vi "FlexMag - 23-03-2023.vi"() -> ()   [LabVIEW 2018] (continued)
                                frame True {
                                n21590 = Wait Until Next ms Multiple(millisecond multiple=u32 200) -> ()  [unwired: 1 out]
                                n21591 = local write "CH3_SoV_Ar_DO"(FALSE ("coating error")) -> ()
                                }
                                }
                                n21592 = local read "coating start"() -> (w25607:bool)
                                n21593 = local read "abort ch3"() -> (w25601:bool)
                                n21594 = Not(x=w25607) -> (.not. x?=w25606:bool)
                                n21595 = Compound Arithmetic op=OR(w25608, w25606, w25601) -> (w25605:bool)
                                }
                                }
                                }
                                }
                                frame True {
                                }
                                }
                                }
                                frame #1 {
                                n21596 = local read "abort ch3"() -> (w25615:bool)
                                n21597 = case shown="False" w25615 {
                                frame False {
                                n21598 = local read "coating start"() -> (w25616:bool)
                                n21599 = case shown="True" w25616 {
                                frame False {
                                }
                                frame True {
                                n21600 = Wait (ms)(milliseconds to wait=u32 100) -> ()  [unwired: 1 out]
                                "coating ch3 led 16" <- TRUE ("coating ch2 led 1")
                                }
                                }
                                }
                                frame True {
                                }
                                }
                                }
                                }
                                }
                                frame #17 {
                                # "BG BV close"
                                n21601 = stacked-sequence {
                                frame #0 {
                                n21602 = local read "abort ch3"() -> (w25619:bool)
                                n21603 = case shown="False" w25619 {
                                frame False {
                                n21604 = local read "coating start"() -> (w25620:bool)
                                n21605 = case shown="True" w25620 {
                                frame False {
                                }
                                frame True {
                                n21606 = while {
                                i -> [w25624]
                                stop <- w25626 stop-if-true
                                n21607 = Greater Or Equal?(x=w25624, y=100) -> (x >= y?=w25625:bool)
                                n21608 = case shown="True" w25625 {
                                frame False {
                                }
                                frame True {
                                n21609 = local write "Warning Message"("Automatic Coating Process is canceled !\nCH3 BG BV couldn't be closed..." ("Warning Message")) -> ()
                                n21610 = local write "coating error"(TRUE ("coating error")) -> ()
                                }
                                }
                                n21611 = local read "CH3_BG_BV_DI"() -> (w25621:bool)
                                n21612 = case shown="True" w25621 {
                                tunnel: [TRUE ("CH2_WFC_DO") FALSE ("CH2_WFC_DO")] -> w25629
                                frame False {
                                }
                                frame True {
                                n21613 = Wait Until Next ms Multiple(millisecond multiple=u32 200) -> ()  [unwired: 1 out]
                                n21614 = local write "CH3_BG_BV_DO"(FALSE ("coating error")) -> ()
                                }
                                }
                                n21615 = local read "coating start"() -> (w25628:bool)
                                n21616 = local read "abort ch3"() -> (w25622:bool)
                                n21617 = Not(x=w25628) -> (.not. x?=w25627:bool)
                                n21618 = Compound Arithmetic op=OR(w25629, w25627, w25622) -> (w25626:bool)
                                }
                                }
                                }
                                }
                                frame True {
                                }
                                }
                                }
                                frame #1 {
                                n21619 = local read "abort ch3"() -> (w25636:bool)
                                n21620 = case shown="False" w25636 {
                                frame False {
                                n21621 = local read "coating start"() -> (w25637:bool)
                                n21622 = case shown="True" w25637 {
                                frame False {
                                }
                                frame True {
                                n21623 = Wait (ms)(milliseconds to wait=u32 100) -> ()  [unwired: 1 out]
                                "coating ch3 led 17" <- TRUE ("coating ch2 led 1")
                                }
                                }
                                }
                                frame True {
                                }
                                }
                                }
                                }
                                }
                                frame #18 {
                                # "CC open"
                                n21624 = stacked-sequence {
                                frame #0 {
                                n21625 = local read "abort ch3"() -> (w25640:bool)
                                n21626 = case shown="False" w25640 {
                                frame False {
                                n21627 = local read "coating start"() -> (w25641:bool)
                                n21628 = case shown="True" w25641 {
                                frame False {
                                }
                                frame True {
                                n21629 = while {
                                i -> [w25645]
                                stop <- w25647 stop-if-true
                                n21630 = Greater Or Equal?(x=w25645, y=100) -> (x >= y?=w25646:bool)
                                n21631 = case shown="True" w25646 {
                                frame False {
                                }
                                frame True {
                                n21632 = local write "Warning Message"("Automatic Coating Process is canceled !\nCH3 CC couldn't be opened..." ("Warning Message")) -> ()
                                n21633 = local write "coating error"(TRUE ("coating error")) -> ()
                                }
                                }
                                n21634 = local read "CH3_CC_DI"() -> (w25642:bool)
                                n21635 = case shown="False" w25642 {
                                tunnel: [FALSE ("CH2_WFC_DO") TRUE ("CH2_WFC_DO")] -> w25650
                                frame False {
                                n21636 = Wait Until Next ms Multiple(millisecond multiple=u32 200) -> ()  [unwired: 1 out]
                                n21637 = local write "CH3_CC_DO"(TRUE ("coating error")) -> ()
                                }
                                frame True {
                                }
                                }
                                n21638 = local read "coating start"() -> (w25649:bool)
                                n21639 = local read "abort ch3"() -> (w25643:bool)
                                n21640 = Not(x=w25649) -> (.not. x?=w25648:bool)
                                n21641 = Compound Arithmetic op=OR(w25650, w25648, w25643) -> (w25647:bool)
                                }
                                }
                                }
                                }
                                frame True {
                                }
                                }
                                }
                                frame #1 {
                                n21642 = local read "abort ch3"() -> (w25657:bool)
                                n21643 = case shown="False" w25657 {
                                frame False {
                                n21644 = local read "coating start"() -> (w25658:bool)
                                n21645 = case shown="True" w25658 {
                                frame False {
                                }
                                frame True {
                                n21646 = Wait (ms)(milliseconds to wait=u32 100) -> ()  [unwired: 1 out]
                                "coating ch3 led 18" <- TRUE ("coating ch2 led 1")
                                }
                                }
                                }
                                frame True {
                                }
                                }
                                }
                                }
                                }
                                frame #19 {
                                # "water close"
                                n21647 = stacked-sequence {
                                frame #0 {
                                n21648 = local read "abort ch3"() -> (w25661:bool)
                                n21649 = case shown="False" w25661 {
                                frame False {
                                n21650 = local read "coating start"() -> (w25662:bool)
                                n21651 = case shown="True" w25662 {
                                frame False {
                                }
                                frame True {
                                n21652 = while {
                                i -> [w25666]
                                stop <- w25668 stop-if-true
                                n21653 = Greater Or Equal?(x=w25666, y=100) -> (x >= y?=w25667:bool)
                                n21654 = case shown="True" w25667 {
                                frame False {
                                }
                                frame True {
                                n21655 = local write "Warning Message"("Automatic Coating Process is canceled !\nCH3 Water Flow couldn't be closed..." ("Warning Message")) -> ()
                                n21656 = local write "coating error"(TRUE ("coating error")) -> ()
                                }
                                }
                                n21657 = local read "CH3_WFC_DI"() -> (w25663:bool)
                                n21658 = case shown="True" w25663 {
                                tunnel: [TRUE ("CH2_WFC_DO") FALSE ("CH2_WFC_DO")] -> w25671
                                frame False {
                                }
                                frame True {
                                n21659 = Wait Until Next ms Multiple(millisecond multiple=u32 200) -> ()  [unwired: 1 out]
                                n21660 = local write "CH3_WFC_DO"(FALSE ("coating error")) -> ()
                                }
                                }
                                n21661 = local read "coating start"() -> (w25670:bool)
                                n21662 = local read "abort ch3"() -> (w25664:bool)
                                n21663 = Not(x=w25670) -> (.not. x?=w25669:bool)
                                n21664 = Compound Arithmetic op=OR(w25671, w25669, w25664) -> (w25668:bool)
                                }
                                }
                                }
                                }
                                frame True {
                                }
                                }
                                }
                                frame #1 {
                                n21665 = local read "abort ch3"() -> (w25678:bool)
                                n21666 = case shown="False" w25678 {
                                frame False {
                                n21667 = local read "coating start"() -> (w25679:bool)
                                n21668 = case shown="True" w25679 {
                                frame False {
                                }
                                frame True {
                                n21669 = Wait (ms)(milliseconds to wait=u32 100) -> ()  [unwired: 1 out]
                                "coating ch3 led 19" <- TRUE ("coating ch2 led 1")
                                }
                                }
                                }
                                frame True {
                                }
                                }
                                }
                                }
                                }
                                frame #20 {
                                # "back roll"
                                n21670 = stacked-sequence {
                                frame #0 {
                                n21671 = local read "abort ch3"() -> (w25682:bool)
                                n21672 = case shown="False" w25682 {
                                frame False {
                                n21673 = local read "coating start"() -> (w25683:bool)
                                n21674 = case shown="True" w25683 {
                                frame False {
                                }
                                frame True {
                                n21675 = disable-structure shown="Enabled" {
                                frame Disabled {
                                n21676 = flat-sequence {
                                frame #0 {
                                n21677 = local read "R DC number steps"() -> (w25684:dbl)
                                n21678 = local write "back roll"(TRUE ("back roll")) -> ()
                                n21679 = local write "step count"(w25684) -> ()
                                }
                                frame #1 {
                                n21680 = Wait (ms)(milliseconds to wait=u32 1000) -> ()  [unwired: 1 out]
                                }
                                frame #2 {
                                n21681 = while {
                                i -> [w25689]
                                stop <- w25695 stop-if-true
                                n21682 = local read "coating start"() -> (w25692:bool)
                                n21683 = local read "back roll"() -> (w25691:bool)
                                n21684 = local read "abort ch3"() -> (w25694:bool)
                                n21685 = Greater?(x=w25689, y=2000) -> (0:w25687:bool)
                                n21686 = local write "coating error"(w25687) -> ()
                                n21687 = Not(x=w25691) -> (.not. x?=w25690:bool)
                                n21688 = Not(x=w25692) -> (.not. x?=w25696:bool)
                                n21689 = Compound Arithmetic op=OR(w25690, w25696, w25694) -> (w25695:bool)
                                n21690 = Wait Until Next ms Multiple(millisecond multiple=u32 200) -> ()  [unwired: 1 out]
                                }
                                }
                                }
                                }
                                frame Enabled {
                                n21691 = local read "dep. for?"() -> (w25698:bool)
                                n21692 = Not(x=w25698) -> (.not. x?=w25699:bool)
                                n21693 = Wait (ms)(milliseconds to wait=u32 100) -> ()  [unwired: 1 out]
                                n21694 = local write "dep. for?"(w25699) -> ()
                                }
                                }
                                }
                                }
                                }
                                frame True {
                                }
                                }
                                }
                                frame #1 {
                                n21695 = local read "abort ch3"() -> (w25700:bool)
                                n21696 = case shown="False" w25700 {
                                frame False {
                                n21697 = local read "coating start"() -> (w25701:bool)
                                n21698 = case shown="True" w25701 {
                                frame False {
                                }
                                frame True {
                                n21699 = Wait (ms)(milliseconds to wait=u32 100) -> ()  [unwired: 1 out]
                                "coating ch3 led 20" <- TRUE ("coating ch2 led 1")
                                }
                                }
                                }
                                frame True {
                                }
                                }
                                }
                                }
                                }
                                frame #21 {
                                # "done"
                                n21700 = stacked-sequence {
                                frame #0 {
                                n21701 = local read "abort ch3"() -> (w25704:bool)
                                n21702 = case shown="False" w25704 {
                                frame False {
                                n21703 = local read "coating start"() -> (w25705:bool)
                                n21704 = case shown="True" w25705 {
                                frame False {
                                }
                                frame True {
                                n21705 = local write "Buzzer DO"(TRUE ("Buzzer DO")) -> ()
                                n21706 = Wait (ms)(milliseconds to wait=u32 3000) -> ()  [unwired: 1 out]
                                n21707 = local write "System Status"("COATING PROCESS DONE (CH3)" ("System Status")) -> ()
                                }
                                }
                                }
                                frame True {
                                }
                                }
                                }
                                frame #1 {
                                n21708 = local read "abort ch3"() -> (w25709:bool)
                                n21709 = case shown="False" w25709 {
                                frame False {
                                n21710 = local read "coating start"() -> (w25710:bool)
                                n21711 = case shown="True" w25710 {
                                frame False {
                                }
                                frame True {
                                n21712 = Wait (ms)(milliseconds to wait=u32 1000) -> ()  [unwired: 1 out]
                                n21713 = local write "System Status"("SEMI-AUTOMATIC MODE " ("System Status")) -> ()
                                n21714 = local write "Buzzer DO"(FALSE ("Buzzer DO")) -> ()
                                }
                                }
                                }
                                frame True {
                                }
                                }
                                }
                                }
                                }
                                }
                                }
                                }
                                }
                              }
                            }
                            frame "rfsputter" {
                              n21715 = disable-structure shown="Enabled" {
                                disable-tunnel: [w25715 TRUE] -> w25714
                                frame Disabled {
                                n21716 = local read "ch4 ch pg torr"() -> (w25720:dbl)
                                n21717 = local read "ch4 cc torr"() -> (w25721:dbl)
                                n21718 = Less Or Equal?(x=w25720, y=0.005) -> (x <= y?=w25719:bool)
                                n21719 = Less Or Equal?(x=w25721, y=0.005) -> (x <= y?=w25718:bool)
                                n21720 = And(x=w25719, y=w25718) -> (x .and. y?=w25715:bool)
                                }
                                frame Enabled {
                                }
                              }
                              n21721 = case shown="True" w25714 {
                                frame False {
                                n21722 = local write "coating error"(TRUE ("coating error")) -> ()
                                n21723 = local write "Warning Message"("Automatic Coating Process is canceled !\nCH4 Pressure should be under 5E-3 Torr .." ("Warning Message")) -> ()
                                }
                                frame True {
                                n21724 = stacked-sequence {
                                frame #0 {
                                }
                                frame #1 {
                                n21725 = stacked-sequence {
                                frame #0 {
                                n21726 = local read "abort ch4"() -> (w25725:bool)
                                n21727 = case shown="False" w25725 {
                                frame False {
                                n21728 = local read "coating start"() -> (w25726:bool)
                                n21729 = case shown="True" w25726 {
                                frame False {
                                }
                                frame True {
                                n21730 = local read "casette_ch4_gui"() -> (w25728:bool)
                                n21731 = Wait (ms)(milliseconds to wait=u32 100) -> ()  [unwired: 1 out]
                                n21732 = case shown="False" w25728 {
                                frame False {
                                n21733 = stacked-sequence {
                                frame #0 {
                                n21734 = flat-sequence {
                                frame #0 {
                                n21735 = local write "target chamber"(4.0 ("target chamber")) -> ()
                                n21736 = Wait (ms)(milliseconds to wait=u32 100) -> ()  [unwired: 1 out]
                                }
                                frame #1 {
                                n21737 = Wait (ms)(milliseconds to wait=u32 1000) -> ()  [unwired: 1 out]
                                }
                                frame #2 {
                                n21738 = local write "transfer vacuum auto"(TRUE ("transfer vacuum")) -> ()
                                }
                                }
                                }
                                frame #1 {
                                n21739 = while {
                                i -> [w25736]
                                stop <- w25738 stop-if-true
                                # "20min"
                                n21740 = local read "present location"() -> (w25742:dbl)
                                n21741 = local read "casette_ch4_gui"() -> (w25734:bool)
                                n21742 = local read "abort ch4"() -> (w25737:bool)
                                n21743 = Equal?(x=w25742, y=4.0) -> (x = y?=w25740:bool)
                                n21744 = Greater?(x=w25736, y=1200) -> (0:w25733:bool)
                                n21745 = local write "trns error"(w25733) -> ()
                                n21746 = Compound Arithmetic op=OR(w25737, w25740, w25734, w25733) -> (w25738:bool)
                                n21747 = Wait Until Next ms Multiple(millisecond multiple=u32 1000) -> ()  [unwired: 1 out]
                                }
                                }
                                }
                                }
                                frame True {
                                }
                                }
                                }
                                }
                                }
                                frame True {
                                }
                                }
                                }
                                frame #1 {
                                n21748 = local read "abort ch4"() -> (w25743:bool)
                                n21749 = case shown="False" w25743 {
                                frame False {
                                n21750 = local read "coating start"() -> (w25744:bool)
                                n21751 = case shown="True" w25744 {
                                frame False {
                                }
                                frame True {
                                n21752 = Wait (ms)(milliseconds to wait=u32 100) -> ()  [unwired: 1 out]
                                n21753 = local write "System Status"("COATING MODE ACTIVE" ("System Status")) -> ()
                                "coating ch4 led 1" <- TRUE ("coating ch2 led 1")
                                }
                                }
                                }
                                frame True {
                                }
                                }
                                }
                                }
                                }
                                frame #2 {
                                # "water"
                                n21754 = stacked-sequence {
                                frame #0 {
                                # "ch1 water off"
                                n21755 = local read "abort ch4"() -> (w25748:bool)
                                n21756 = case shown="False" w25748 {
                                frame False {
                                n21757 = local read "coating start"() -> (w25749:bool)
                                n21758 = case shown="True" w25749 {
                                frame False {
                                }
                                frame True {
                                n21759 = while {
                                i -> [w25752]
                                stop <- w25754 stop-if-true
                                n21760 = Greater Or Equal?(x=w25752, y=100) -> (x >= y?=w25753:bool)
                                n21761 = case shown="True" w25753 {
                                frame False {
                                }
                                frame True {
                                n21762 = local write "coating error"(TRUE ("coating error")) -> ()
                                n21763 = local write "Warning Message"("Automatic Coating Process is canceled !\nCH1 Water Flow Problem.." ("Warning Message")) -> ()
                                }
                                }
                                n21764 = local read "CH1_WFC_DI"() -> (w25758:bool)
                                n21765 = case shown="True" w25758 {
                                tunnel: [TRUE ("CH2_WFC_DO") FALSE ("CH2_WFC_DO")] -> w25757
                                frame False {
                                }
                                frame True {
                                n21766 = Wait Until Next ms Multiple(millisecond multiple=u32 200) -> ()  [unwired: 1 out]
                                n21767 = local write "CH1_WFC_DO"(FALSE ("CH2_WFC_DO")) -> ()
                                }
                                }
                                n21768 = local read "coating start"() -> (w25756:bool)
                                n21769 = local read "abort ch4"() -> (w25750:bool)
                                n21770 = Not(x=w25756) -> (.not. x?=w25755:bool)
                                n21771 = Compound Arithmetic op=OR(w25757, w25755, w25750) -> (w25754:bool)
                                }
                                }
                                }
                                }
                                frame True {
                                }
                                }
                                }
                                frame #1 {
                                # "ch3 water off"
                                n21772 = local read "abort ch4"() -> (w25765:bool)
                                n21773 = case shown="False" w25765 {
                                frame False {
                                n21774 = local read "coating start"() -> (w25766:bool)
                                n21775 = case shown="True" w25766 {
                                frame False {
                                }
                                frame True {
                                n21776 = while {
                                i -> [w25769]
                                stop <- w25771 stop-if-true
                                n21777 = Greater Or Equal?(x=w25769, y=100) -> (x >= y?=w25770:bool)
                                n21778 = case shown="True" w25770 {
                                frame False {
                                }
                                frame True {
                                n21779 = local write "coating error"(TRUE ("coating error")) -> ()
                                n21780 = local write "Warning Message"("Automatic Coating Process is canceled !\nCH3 Water Flow Problem.." ("Warning Message")) -> ()
                                }
                                }
                                n21781 = local read "CH3_WFC_DI"() -> (w25775:bool)
                                n21782 = case shown="True" w25775 {
                                tunnel: [TRUE ("CH2_WFC_DO") FALSE ("CH2_WFC_DO")] -> w25774
                                frame False {
                                }
                                frame True {
                                n21783 = Wait Until Next ms Multiple(millisecond multiple=u32 200) -> ()  [unwired: 1 out]
                                n21784 = local write "CH3_WFC_DO"(FALSE ("CH2_WFC_DO")) -> ()
                                }
                                }
                                n21785 = local read "coating start"() -> (w25773:bool)
                                n21786 = local read "abort ch4"() -> (w25767:bool)
                                n21787 = Not(x=w25773) -> (.not. x?=w25772:bool)
                                n21788 = Compound Arithmetic op=OR(w25774, w25772, w25767) -> (w25771:bool)
                                }
                                }
                                }
                                }
                                frame True {
                                }
                                }
                                }
                                frame #2 {
                                # "ch2 water off"
                                n21789 = local read "abort ch4"() -> (w25782:bool)
                                n21790 = case shown="False" w25782 {
                                frame False {
                                n21791 = local read "coating start"() -> (w25783:bool)
                                n21792 = case shown="True" w25783 {
                                frame False {
                                }
                                frame True {
                                n21793 = while {
                                i -> [w25786]
                                stop <- w25788 stop-if-true
                                n21794 = Greater Or Equal?(x=w25786, y=100) -> (x >= y?=w25787:bool)
                                n21795 = case shown="True" w25787 {
                                frame False {
                                }
                                frame True {
                                n21796 = local write "coating error"(TRUE ("coating error")) -> ()
                                n21797 = local write "Warning Message"("Automatic Coating Process is canceled !\nCH2 Water Flow Problem.." ("Warning Message")) -> ()
                                }
                                }
                                n21798 = local read "CH2_WFC_DI"() -> (w25792:bool)
                                n21799 = case shown="True" w25792 {
                                tunnel: [TRUE ("CH2_WFC_DO") FALSE ("CH2_WFC_DO")] -> w25791
                                frame False {
                                }
                                frame True {
                                n21800 = Wait Until Next ms Multiple(millisecond multiple=u32 200) -> ()  [unwired: 1 out]
                                n21801 = local write "CH2_WFC_DO"(FALSE ("CH2_WFC_DO")) -> ()
                                }
                                }
                                n21802 = local read "coating start"() -> (w25790:bool)
                                n21803 = local read "abort ch4"() -> (w25784:bool)
                                n21804 = Not(x=w25790) -> (.not. x?=w25789:bool)
                                n21805 = Compound Arithmetic op=OR(w25791, w25789, w25784) -> (w25788:bool)
                                }
                                }
                                }
                                }
                                frame True {
                                }
                                }
                                }
                                frame #3 {
                                # "ch4 water on"
                                n21806 = local read "abort ch4"() -> (w25799:bool)
                                n21807 = case shown="False" w25799 {
                                frame False {
                                n21808 = local read "coating start"() -> (w25800:bool)
                                n21809 = case shown="True" w25800 {
                                frame False {
                                }
                                frame True {
                                n21810 = while {
                                i -> [w25803]
                                stop <- w25805 stop-if-true
                                n21811 = Greater Or Equal?(x=w25803, y=100) -> (x >= y?=w25804:bool)
                                n21812 = case shown="True" w25804 {
                                frame False {
                                }
                                frame True {
                                n21813 = local write "coating error"(TRUE ("coating error")) -> ()
                                n21814 = local write "Warning Message"("Automatic Coating Process is canceled !\nCH4 Water Flow Problem.." ("Warning Message")) -> ()
                                }
                                }
                                n21815 = local read "CH4_WFC_DI"() -> (w25809:bool)
                                n21816 = case shown="False" w25809 {
                                tunnel: [FALSE ("CH2_WFC_DO") TRUE ("CH2_WFC_DO")] -> w25808
                                frame False {
                                n21817 = Wait Until Next ms Multiple(millisecond multiple=u32 200) -> ()  [unwired: 1 out]
                                n21818 = local write "CH4_WFC_DO"(TRUE ("CH2_WFC_DO")) -> ()
                                }
                                frame True {
                                }
                                }
                                n21819 = local read "coating start"() -> (w25807:bool)
                                n21820 = local read "abort ch4"() -> (w25801:bool)
                                n21821 = Not(x=w25807) -> (.not. x?=w25806:bool)
                                n21822 = Compound Arithmetic op=OR(w25808, w25806, w25801) -> (w25805:bool)
                                }
                                }
                                }
                                }
                                frame True {
                                }
                                }
                                }
                                frame #4 {
                                n21823 = local read "abort ch4"() -> (w25816:bool)
                                n21824 = case shown="False" w25816 {
                                frame False {
                                n21825 = local read "coating start"() -> (w25817:bool)
                                n21826 = case shown="True" w25817 {
                                frame False {
                                }
                                frame True {
                                n21827 = Wait (ms)(milliseconds to wait=u32 100) -> ()  [unwired: 1 out]
                                "coating ch4 led 2" <- TRUE ("coating ch2 led 1")
                                }
                                }
                                }
                                frame True {
                                }
                                }
                                }
                                }
                                }
                                frame #3 {
                                # "ch2 pcgv on"
                                n21828 = stacked-sequence {
                                frame #0 {
                                n21829 = local read "abort ch4"() -> (w25820:bool)
                                n21830 = case shown="False" w25820 {
                                frame False {
                                n21831 = local read "coating start"() -> (w25821:bool)
                                n21832 = case shown="True" w25821 {
                                frame False {
                                }
                                frame True {
                                n21833 = local read "ch4_pcgv_gui"() -> (w25822:bool)
                                n21834 = case shown="False" w25822 {
                                frame False {
                                n21835 = flat-sequence {
                                frame #0 {
                                n21836 = local write "pcgv4 auto open"(TRUE ("pcgv2 auto open")) -> ()
                                }
                                frame #1 {
                                n21837 = Wait (ms)(milliseconds to wait=u32 1000) -> ()  [unwired: 1 out]
                                }
                                frame #2 {
                                n21838 = local write "pcgv4 auto open"(TRUE ("pcgv2 auto open")) -> ()
                                }
                                }
                                }
                                frame True {
                                }
                                }
                                }
                                }
                                }
                                frame True {
                                }
                                }
                                }
                                frame #1 {
                                n21839 = local read "abort ch4"() -> (w25826:bool)
                                n21840 = case shown="False" w25826 {
                                frame False {
                                n21841 = local read "coating start"() -> (w25827:bool)
                                n21842 = case shown="True" w25827 {
                                frame False {
                                }
                                frame True {
                                n21843 = while {
                                i -> [w25830]
                                stop <- w25832 stop-if-true
                                n21844 = Greater Or Equal?(x=w25830, y=100) -> (x >= y?=w25831:bool)
                                n21845 = case shown="True" w25831 {
                                frame False {
                                }
                                frame True {
                                n21846 = local write "coating error"(TRUE ("coating error")) -> ()
                                n21847 = local write "Warning Message"("Automatic Coating Process is canceled !\nCH4 PCGV couldn't be opened.." ("Warning Message")) -> ()
                                }
                                }
                                n21848 = local read "ch4_pcgv_gui"() -> (w25836:bool)
                                n21849 = case shown="True" w25836 {
                                tunnel: [FALSE ("CH2_WFC_DO") TRUE ("CH2_WFC_DO")] -> w25835
                                frame False {
                                n21850 = Wait Until Next ms Multiple(millisecond multiple=u32 200) -> ()  [unwired: 1 out]
                                }
                                frame True {
                                }
                                }
                                n21851 = local read "coating start"() -> (w25834:bool)
                                n21852 = local read "abort ch4"() -> (w25828:bool)
                                n21853 = Not(x=w25834) -> (.not. x?=w25833:bool)
                                n21854 = Compound Arithmetic op=OR(w25835, w25833, w25828) -> (w25832:bool)
                                }
                                }
                                }
                                }
                                frame True {
                                }
                                }
                                }
                                frame #2 {
                                n21855 = local read "abort ch4"() -> (w25842:bool)
                                n21856 = case shown="False" w25842 {
                                frame False {
                                n21857 = local read "coating start"() -> (w25843:bool)
                                n21858 = case shown="True" w25843 {
                                frame False {
                                }
                                frame True {
                                n21859 = Wait (ms)(milliseconds to wait=u32 100) -> ()  [unwired: 1 out]
                                "coating ch4 led 3" <- TRUE ("coating ch2 led 1")
                                }
                                }
                                }
                                frame True {
                                }
                                }
                                }
                                }
                                }
                                frame #4 {
                                # "RF host - communication check"
                                n21860 = stacked-sequence {
                                frame #0 {
                                n21861 = local read "abort ch4"() -> (w25846:bool)
                                n21862 = case shown="False" w25846 {
                                frame False {
                                n21863 = local read "coating start"() -> (w25847:bool)
                                n21864 = case shown="True" w25847 {
                                frame False {
                                }
                                frame True {
                                n21865 = flat-sequence {
                                frame #0 {
                                n21866 = local write "RF_auto_host"(TRUE ("pcgv2 auto open")) -> ()
                                }
                                frame #1 {
                                n21867 = Wait (ms)(milliseconds to wait=u32 5000) -> ()  [unwired: 1 out]
                                }
                                frame #2 {
                                n21868 = local write "RF_auto_host"(TRUE ("pcgv2 auto open")) -> ()
                                }
                                }
                                }
                                }
                                }
                                frame True {
                                }
                                }
                                }
                                frame #1 {
                                n21869 = local read "abort ch4"() -> (w25851:bool)
                                n21870 = case shown="False" w25851 {
                                frame False {
                                n21871 = local read "coating start"() -> (w25852:bool)
                                n21872 = case shown="True" w25852 {
                                frame False {
                                }
                                frame True {
                                n21873 = disable-structure shown="Disabled" {
                                frame Disabled {
                                n21874 = while {
                                i -> [w25855]
                                stop <- w25857 stop-if-true
                                n21875 = Greater Or Equal?(x=w25855, y=100) -> (x >= y?=w25856:bool)
                                n21876 = case shown="True" w25856 {
                                frame False {
                                }
                                frame True {
                                n21877 = local write "coating error"(TRUE ("coating error")) -> ()
                                n21878 = local write "Warning Message"("Automatic Coating Process is canceled !\nDCPS Problem.." ("Warning Message")) -> ()
                                }
                                }
                                n21879 = local read "Dcps_fail"() -> (w25861:bool)
                                n21880 = case shown="True" w25861 {
                                tunnel: [TRUE ("CH2_WFC_DO") FALSE ("CH2_WFC_DO")] -> w25860
                                frame False {
                                }
                                frame True {
                                n21881 = Wait Until Next ms Multiple(millisecond multiple=u32 200) -> ()  [unwired: 1 out]
                                }
                                }
                                n21882 = local read "coating start"() -> (w25859:bool)
                                n21883 = local read "abort ch4"() -> (w25853:bool)
                                n21884 = Not(x=w25859) -> (.not. x?=w25858:bool)
                                n21885 = Compound Arithmetic op=OR(w25860, w25858, w25853) -> (w25857:bool)
                                }
                                }
                                frame Enabled {
                                }
                                }
                                }
                                }
                                }
                                frame True {
                                }
                                }
                                }
                                frame #2 {
                                n21886 = local read "abort ch4"() -> (w25867:bool)
                                n21887 = case shown="False" w25867 {
                                frame False {
                                n21888 = local read "coating start"() -> (w25868:bool)
                                n21889 = case shown="True" w25868 {
                                frame False {
                                }
                                frame True {
                                n21890 = Wait (ms)(milliseconds to wait=u32 100) -> ()  [unwired: 1 out]
                                "coating ch4 led 4" <- TRUE ("coating ch2 led 1")
                                }
                                }
                                }
                                frame True {
                                }
                                }
                                }
                                }
                                }
                                frame #5 {
                                # "magnetron selection"
                                n21891 = disable-structure shown="Disabled" {
                                frame Disabled {
                                n21892 = stacked-sequence {
                                frame #0 {
                                n21893 = local read "abort ch4"() -> (w25871:bool)
                                n21894 = case shown="False" w25871 {
                                frame False {
                                n21895 = local read "coating start"() -> (w25872:bool)
                                n21896 = case shown="True" w25872 {
                                frame False {
                                }
                                frame True {
                                n21897 = local write "DCPS_ SW2 DO"(FALSE ("pcgv2 auto open")) -> ()
                                n21898 = local write "DCPS_ SW1 DO"(TRUE ("pcgv2 auto open")) -> ()
                                n21899 = Wait (ms)(milliseconds to wait=u32 1000) -> ()  [unwired: 1 out]
                                }
                                }
                                }
                                frame True {
                                }
                                }
                                }
                                frame #1 {
                                n21900 = local read "abort ch4"() -> (w25876:bool)
                                n21901 = case shown="False" w25876 {
                                frame False {
                                n21902 = local read "coating start"() -> (w25877:bool)
                                n21903 = case shown="True" w25877 {
                                frame False {
                                }
                                frame True {
                                n21904 = while {
                                i -> [w25880]
                                stop <- w25882 stop-if-true
                                n21905 = Greater Or Equal?(x=w25880, y=100) -> (x >= y?=w25881:bool)
                                n21906 = case shown="True" w25881 {
                                frame False {
                                }
                                frame True {
                                n21907 = local write "Warning Message"("Automatic Coating Process is canceled !\nDCPS Magnetron Selection Problem.." ("Warning Message")) -> ()
                                n21908 = local write "coating error"(TRUE ("coating error")) -> ()
                                }
                                }
                                n21909 = local read "DCPS_ SW1 DI"() -> (w25886:bool)
                                n21910 = case shown="False" w25886 {
                                tunnel: [FALSE ("CH2_WFC_DO") TRUE ("CH2_WFC_DO")] -> w25885
                                frame False {
                                n21911 = local write "DCPS_ SW1 DO"(TRUE ("CH2_WFC_DO")) -> ()
                                n21912 = local write "DCPS_ SW2 DO"(FALSE ("CH2_WFC_DO")) -> ()
                                n21913 = Wait Until Next ms Multiple(millisecond multiple=u32 200) -> ()  [unwired: 1 out]
                                }
                                frame True {
                                }
                                }
                                n21914 = local read "coating start"() -> (w25884:bool)
                                n21915 = local read "abort ch2"() -> (w25878:bool)
                                n21916 = Not(x=w25884) -> (.not. x?=w25883:bool)
                                n21917 = Compound Arithmetic op=OR(w25885, w25883, w25878) -> (w25882:bool)
                                }
                                }
                                }
                                }
                                frame True {
                                }
                                }
                                }
                                frame #2 {
                                n21918 = local read "abort ch2"() -> (w25894:bool)
                                n21919 = case shown="False" w25894 {
                                frame False {
                                n21920 = local read "coating start"() -> (w25895:bool)
                                n21921 = case shown="True" w25895 {
                                frame False {
                                }
                                frame True {
                                n21922 = Wait (ms)(milliseconds to wait=u32 100) -> ()  [unwired: 1 out]
                                "coating ch4 led 5" <- TRUE ("coating ch2 led 1")
                                }
                                }
                                }
                                frame True {
                                }
                                }
                                }
                                }
                                }
                                frame Enabled {
                                }
                                }
                                }
                                frame #6 {
                                # "cc close"
                                n21923 = stacked-sequence {
                                frame #0 {
                                n21924 = local read "abort ch4"() -> (w25898:bool)
                                n21925 = case shown="False" w25898 {
                                frame False {
                                n21926 = local read "coating start"() -> (w25899:bool)
                                n21927 = case shown="True" w25899 {
                                frame False {
                                }
                                frame True {
                                n21928 = while {
                                i -> [w25902]
                                stop <- w25904 stop-if-true
                                n21929 = Greater Or Equal?(x=w25902, y=100) -> (x >= y?=w25903:bool)
                                n21930 = case shown="True" w25903 {
                                frame False {
                                }
                                frame True {
                                n21931 = local write "Warning Message"("Automatic Coating Process is canceled !\nCH4 ColdCathode couldn't be closed.." ("Warning Message")) -> ()
                                n21932 = local write "coating error"(TRUE ("coating error")) -> ()
                                }
                                }
                                n21933 = local read "CH4_CC_DI"() -> (w25908:bool)
                                n21934 = case shown="True" w25908 {
                                tunnel: [TRUE ("CH2_WFC_DO") FALSE ("CH2_WFC_DO")] -> w25907
                                frame False {
                                }
                                frame True {
                                n21935 = Wait Until Next ms Multiple(millisecond multiple=u32 200) -> ()  [unwired: 1 out]
                                n21936 = local write "CH4_CC_DO"(FALSE ("coating error")) -> ()
                                }
                                }
                                n21937 = local read "coating start"() -> (w25906:bool)
                                n21938 = local read "abort ch4"() -> (w25900:bool)
                                n21939 = Not(x=w25906) -> (.not. x?=w25905:bool)
                                n21940 = Compound Arithmetic op=OR(w25907, w25905, w25900) -> (w25904:bool)
                                }
                                }
                                }
                                }
                                frame True {
                                }
                                }
                                }
                                frame #1 {
                                n21941 = local read "abort ch4"() -> (w25915:bool)
                                n21942 = case shown="False" w25915 {
                                frame False {
                                n21943 = local read "coating start"() -> (w25916:bool)
                                n21944 = case shown="True" w25916 {
                                frame False {